vi "datataker.vi"() -> ()   [LabVIEW 2012]
doc: "This example demonstrates how to acquire a single buffer of voltage measurements using a DAQmx device.\n\nFor instructions on how to connect your signals to the DAQ device, refer to your device documentation."
uses:
  <vilib>/userdefined/High Color/nirio_resource_hc.ctl
  <vilib>/Utility/error.llb/DialogType.ctl
  <vilib>/FPGAPlugInAG/PCIe-7841R/niLvFpga_Open_PCIe-7841R.vi
  <vilib>/DAQmx/create/channels.llb/DAQmx Create Channel (AI-Voltage-Basic).vi
  <vilib>/DAQmx/configure/timing.llb/DAQmx Timing (Sample Clock).vi
  <vilib>/DAQmx/configure/trigger.llb/DAQmx Start Trigger (Digital Edge).vi
  <vilib>/rvi/interface/nirviOpenFPGA/nirviOpenFPGA.xnode
  fpga/MultiChannelFeed_FPGATarget2_feedbackcooling(_T5hmXv3JUos.lvbitx
  <resource>/objmgr/daqmx.rc
panel:
  in  "sweep time (S)":ext=10.0 format="%.2f"
  in  "sweep stop (Hz)":ext=200.0
  in  "sweep start (Hz)":ext=1.0
  in  "chirp?":bool
  in  "stop (F)":ext=200.0
  in  "start (F)":ext=10.0
  in  "Number of F Steps":i32=20
  in  "dc offset?":bool=TRUE
  in  "volt_div":dbl=200.0
  in  "Set synth?":bool=TRUE
  in  "stop (V)":ext=2.5
  in  "start (V)":ext=2.5
  in  "Number of V Steps":i32=1
  out "error out":errorcluster
  in  "Physical Channel (drive signals)":tag="Dev5/ai0"
  out "Curr threshold":dbl
  in  "Stop threshold":dbl=0.05
  in  "Stop flashing below thresh":bool
  out "Pirani pressure (mbar)":string="0000\r\n"
  out "CC read error":errorcluster={"status"=FALSE, "code"=1073676294, "source"="VISA Read in read_pressure(SubVI).vi->hdf5(SubVI).vi->datataker.vi"}
  out "CC pressure (mbar)":string="4."
  out "Pirani read error":errorcluster={"status"=FALSE, "code"=1073676294, "source"="VISA Read in read_pressure(SubVI).vi->hdf5(SubVI).vi->datataker.vi"}
  in  "# Pulses":i32=3
  in  "Output channel (for flashing)":tag="Dev4/ao0"
  in  "Number of cyles\nbetween flashes":i32=3
  in  "Flash lamp?":bool
  in  "File base name":string="5e-7mbar_xyzcool"
  in  "Delay time between files(s)":dbl caption="Delay Time (s)"
  in  "Num files":i32=100000
  out "Temps (C):":dbl[](array[numeric])=[24.1, 24.6]
  in  "VISA Refnum in":refnum<visa-resource-name>="GPIB0::19::INSTR"
  in  "RIO Device":T1="RIO0::INSTR"
  in  "Directory path":path=path "D:/Data/20140623/Bead1/freq_sweep_finer"
  out "Waveform Graph":dbl[][](graph)
  in  "Number of Samples":i32=500000
  in  "Sample Rate":dbl=5000.0
  in  "Sample Clock Source":tag="/Dev2/PXI_Clk10"
  in  "Terminal Configuration":i32(ring)=-1 items=["default"=-1, "RSE"=10083, "NRSE"=10078, "Differential"=10106, "Pseudodifferential"=12529]
  in  "Max Voltage":dbl=10.0
  in  "Physical Channels (Position signals)":tag="Dev2/ai0:7"
  out "Actual Sample Rate":dbl=5000.0 format="%0.2f"
  # "Channel Settings"
  # "Acquired Data"
  # "Timing Settings"
  # "Flash Lamp Settings"
  # "Pressures and Temperatures"
  # "Logging Settings"
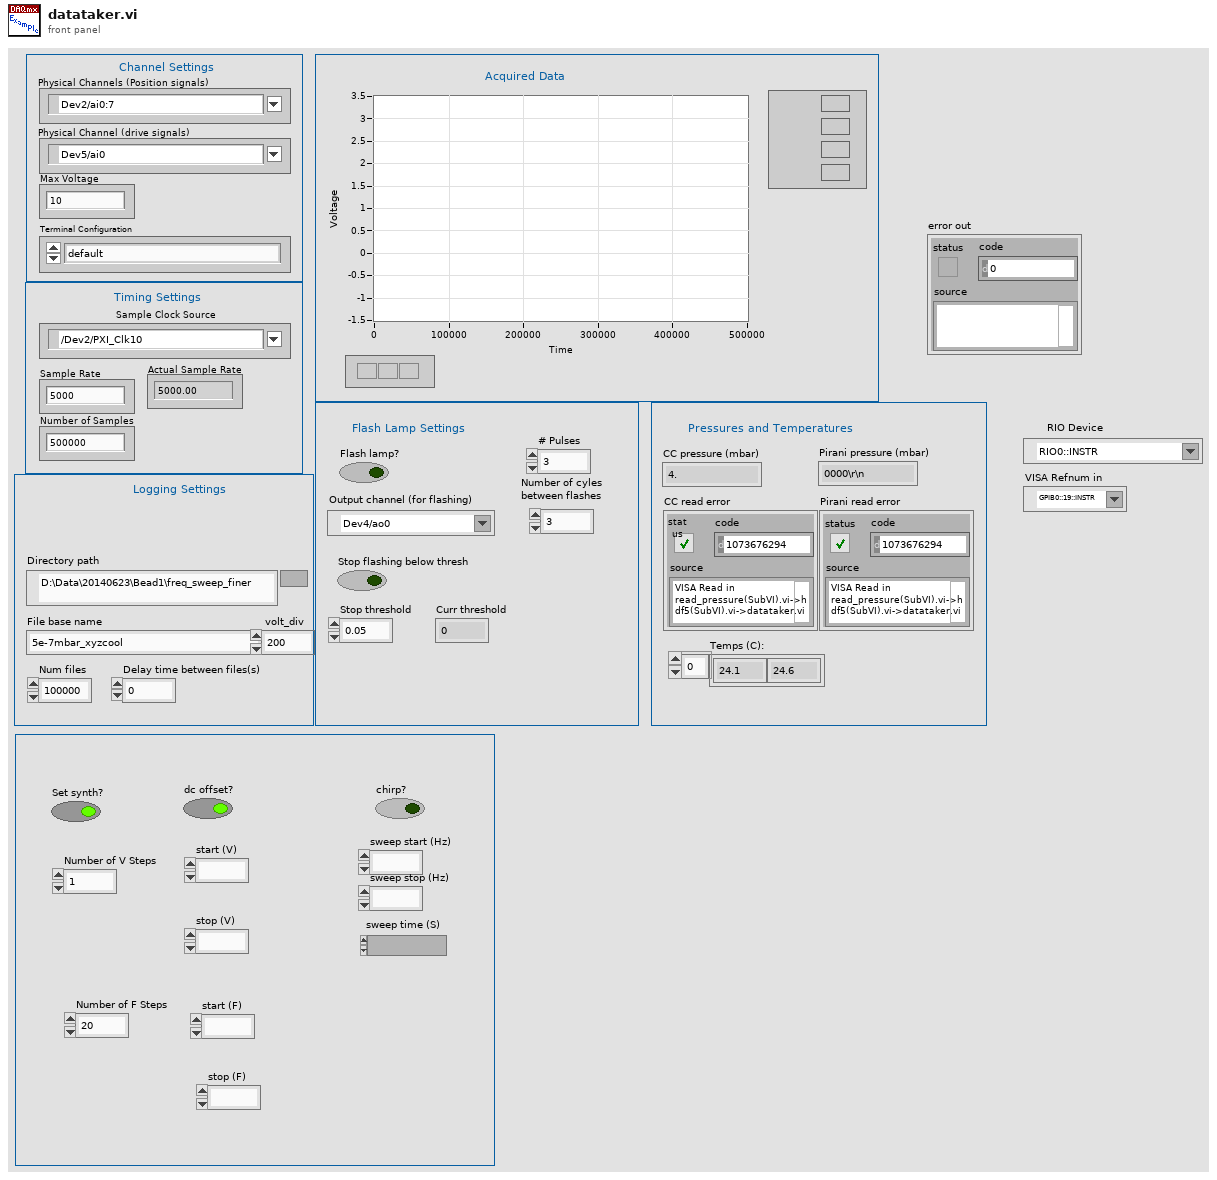
[diagram p1: front panel]
types:
  T1 = typedef "nirio_resource_hc.ctl" = tag
  T2 = typedef "DialogType.ctl" = u16
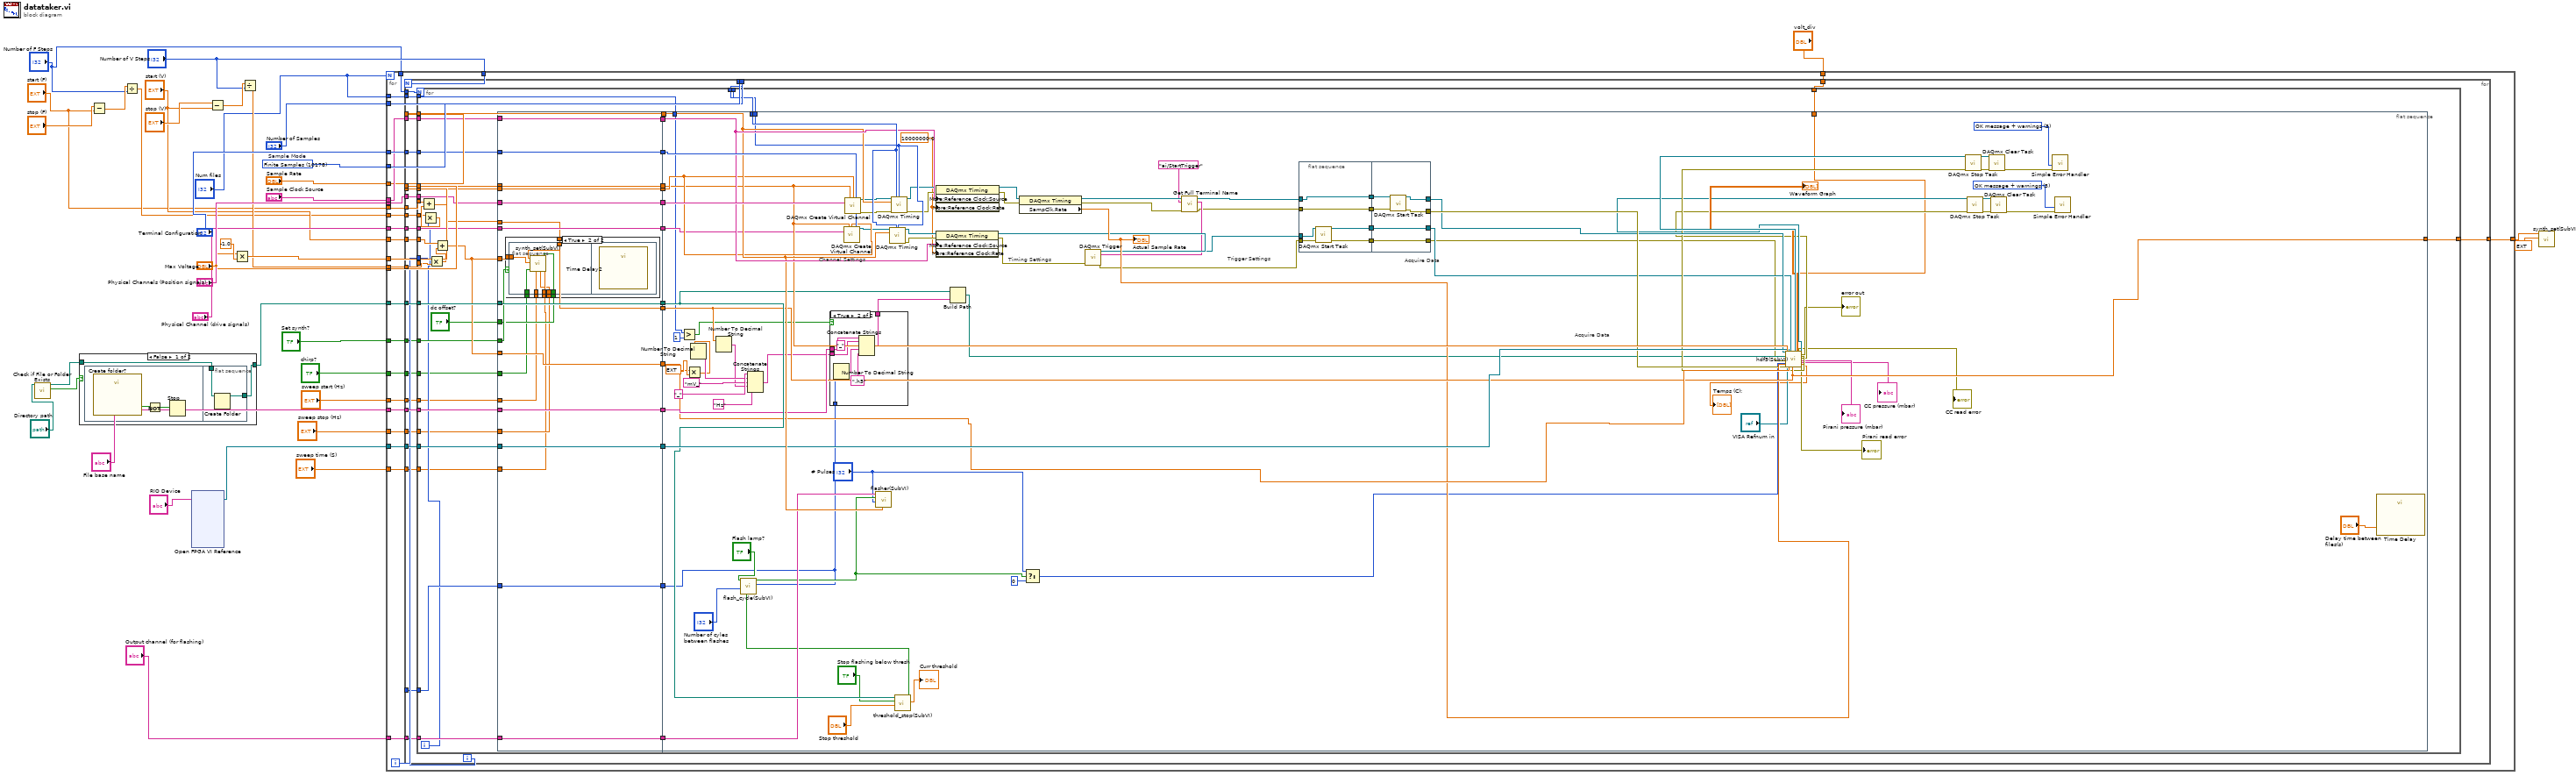
[diagram p0: block diagram]
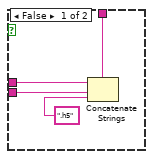
[diagram p3: hidden frame]
diagram:
  w37 = 10178 items=["Finite Samples"=10178, "Continuous Samples"=10123, "Hardware Timed Single Point"=12522]  # Sample Mode
  n1 = call <vilib>:"Check if File or Folder Exists.vi"("path"="Directory path") -> ("file or folder exists?"=w25:bool, "dup path"=w24:path)  [unwired: 8 in, 1 out]
  n2 = case shown="False" w25 {
    tunnel: w24 -> [w39 w44]
    tunnel: [w38 w44] -> w23
    frame False {
      n3 = flat-sequence {
        tunnel: w39 -> [w43]
        tunnel: [w42] -> w38
        frame #0 {
          n4 = call "Create folder?"() -> ("OK"=w41:bool)  [unwired: 18 in, 1 out]
          n5 = Not(x=w41) -> (.not. x?=w40:bool)
          n6 = Stop(stop? (T)=w40) -> ()
        }
        frame #1 {
          n7 = Create Folder(path (use dialog)=w43) -> (created path=w42:path)  [unwired: 2 in, 2 out]
        }
      }
    }
    frame True {
    }
  }
  n8 = Subtract(x="stop (F)", y="start (F)") -> (x-y=w9:ext)
  n9 = Divide(x=w9, y="Number of F Steps") -> (x/y=w8:ext)
  n10 = xnode "Open FPGA VI Reference"("resource name"="RIO Device") -> ("FPGA VI Reference Out"=w27:refnum<k20>)  [unwired: 1 in, 1 out]
  n11 = Subtract(x="stop (V)", y="start (V)") -> (x-y=w18:ext)
  n12 = Multiply(x="Max Voltage", y=-1.0) -> (x*y=w30:dbl)
  n13 = Divide(x=w18, y="Number of V Steps") -> (x/y=w16:ext)
  n14 = for {
    N: "Num files" -> [_]
    tunnel: w37 -> [w72]
    tunnel: "Physical Channels (Position signals)" -> [w71]
    tunnel: "Terminal Configuration" -> [w70]
    tunnel: "Sample Clock Source" -> [w69]
    tunnel: "Sample Rate" -> [w68]
    tunnel: "Number of Samples" -> [w67]
    tunnel: w30 -> [w66]
    tunnel: "Max Voltage" -> [w65]
    tunnel: w27 -> [w64]
    tunnel: w23 -> [w63]
    tunnel: "File base name" -> [w62]
    tunnel: "Output channel (for flashing)" -> [w61]
    tunnel: "Physical Channel (drive signals)" -> [w60]
    tunnel: "Number of V Steps" -> [w59]
    tunnel: w16 -> [w58]
    tunnel: "start (V)" -> [w57]
    tunnel: [w56] -> w6
    tunnel: "Num files" -> [w54]
    tunnel: "Set synth?" -> [w53]
    tunnel: "volt_div" -> [w52]
    tunnel: w8 -> [w51]
    tunnel: "start (F)" -> [w50]
    tunnel: "Number of F Steps" -> [w49]
    tunnel: "chirp?" -> [w48]
    tunnel: "sweep start (Hz)" -> [w47]
    tunnel: "sweep stop (Hz)" -> [w46]
    tunnel: "sweep time (S)" -> [w45]
    i -> [w55]
    n15 = for {
      N: w59 -> [_]
      tunnel: w72 -> [w100]
      tunnel: w71 -> [w99]
      tunnel: w70 -> [w98]
      tunnel: w69 -> [w97]
      tunnel: w68 -> [w96]
      tunnel: w67 -> [w95]
      tunnel: w66 -> [w94]
      tunnel: w65 -> [w93]
      tunnel: w64 -> [w92]
      tunnel: w63 -> [w91]
      tunnel: w62 -> [w90]
      tunnel: w61 -> [w89]
      tunnel: w60 -> [w88]
      tunnel: w58 -> [w87]
      tunnel: w57 -> [w86]
      tunnel: [w85] -> w56
      tunnel: w55 -> [w83]
      tunnel: w54 -> [w82]
      tunnel: w53 -> [w81]
      tunnel: w52 -> [w80]
      tunnel: w51 -> [w79]
      tunnel: w50 -> [w78]
      tunnel: w49 -> [w77]
      tunnel: w48 -> [w76]
      tunnel: w47 -> [w75]
      tunnel: w46 -> [w74]
      tunnel: w45 -> [w73]
      i -> [w84]
      n16 = for {
        N: w77 -> [_]
        tunnel: w100 -> [w133]
        tunnel: w99 -> [w132]
        tunnel: w98 -> [w131]
        tunnel: w97 -> [w130]
        tunnel: w96 -> [w129]
        tunnel: w95 -> [w128]
        tunnel: w94 -> [w127]
        tunnel: w93 -> [w126]
        tunnel: w92 -> [w125]
        tunnel: w91 -> [w124]
        tunnel: w90 -> [w123]
        tunnel: w89 -> [w122]
        tunnel: w88 -> [w121]
        tunnel: w87 -> [w120]
        tunnel: w86 -> [w118]
        tunnel: [w116] -> w85
        tunnel: w84 -> [w115]
        tunnel: w83 -> [w114]
        tunnel: w82 -> [w113]
        tunnel: w81 -> [w112]
        tunnel: w80 -> [w111]
        tunnel: w79 -> [w107]
        tunnel: w78 -> [w106]
        tunnel: w76 -> [w104]
        tunnel: w75 -> [w103]
        tunnel: w74 -> [w102]
        tunnel: w73 -> [w101]
        i -> [w105]
        n17 = Multiply(x=w107, y=w105) -> (x*y=w108:ext)
        n18 = Add(x=w106, y=w108) -> (x+y=w109:ext)
        n19 = Multiply(x=w115, y=w120) -> (x*y=w119:ext)
        n20 = Add(x=w118, y=w119) -> (x+y=w117:ext)
        n21 = flat-sequence {
          tunnel: w121 -> [w157]
          tunnel: w122 -> [w158]
          tunnel: w123 -> [w159]
          tunnel: w124 -> [w160]
          tunnel: w125 -> [w161]
          tunnel: w126 -> [w162]
          tunnel: w127 -> [w163]
          tunnel: w130 -> [w164]
          tunnel: w131 -> [w165]
          tunnel: w132 -> [w166]
          tunnel: [w166] -> w146
          tunnel: [w165] -> w145
          tunnel: [w164] -> w144
          tunnel: [w163] -> w143
          tunnel: [w162] -> w142
          tunnel: [w161] -> w141
          tunnel: [w160] -> w140
          tunnel: [w159] -> w139
          tunnel: [w158] -> w138
          tunnel: [w157] -> w137
          tunnel: w109 -> [w155]
          tunnel: w117 -> [w156]
          tunnel: [w155] -> w136
          tunnel: w117 -> [w154]
          tunnel: [w154] -> w135
          tunnel: w114 -> [w153]
          tunnel: [w153] -> w134
          tunnel: w112 -> [w152]
          tunnel: "dc offset?" -> [w151]
          tunnel: w104 -> [w150]
          tunnel: w103 -> [w149]
          tunnel: w102 -> [w148]
          tunnel: w101 -> [w147]
          tunnel: w133 -> [w270]
          tunnel: w129 -> [w266]
          tunnel: w128 -> [w265]
          tunnel: w146 -> [w269]
          tunnel: w145 -> [w268]
          tunnel: w144 -> [w267]
          tunnel: w143 -> [w264]
          tunnel: w142 -> [w263]
          tunnel: w141 -> [w262]
          tunnel: w140 -> [w261]
          tunnel: w139 -> [w260]
          tunnel: w138 -> [w259]
          tunnel: w137 -> [w258]
          tunnel: w136 -> [w256]
          tunnel: w135 -> [w257]
          tunnel: [w256] -> w116
          tunnel: w134 -> [w183]
          tunnel: w113 -> [w182]
          tunnel: w111 -> [w181]
          frame #0 {
            n22 = case shown="True" w152 {
              tunnel: w156 -> [_ w173]
              tunnel: w155 -> [_ w172]
              tunnel: w151 -> [_ w171]
              tunnel: w150 -> [_ w170]
              tunnel: w149 -> [_ w169]
              tunnel: w148 -> [_ w168]
              tunnel: w147 -> [_ w167]
              frame False {
              }
              frame True {
                n23 = flat-sequence {
                  tunnel: w173 -> [w180]
                  tunnel: w172 -> [w179]
                  tunnel: w171 -> [w178]
                  tunnel: w170 -> [w177]
                  tunnel: w169 -> [w176]
                  tunnel: w168 -> [w174]
                  tunnel: w167 -> [w175]
                  frame #0 {
                    n24 = call "synth_set(SubVI).vi"("sweep time (S)"=w175, "dc offset?"=w178, "sweep stop (Hz)"=w174, "sweep start (Hz)"=w176, "chirp?"=w177, "amplitude (V)"=w180, "frequency (Hz)"=w179) -> ()  [unwired: 5 in]
                  }
                  frame #1 {
                    n25 = call "Time Delay2"() -> ()  [unwired: 11 in, 1 out]
                  }
                }
              }
            }
          }
          frame #1 {
            w201 = 10000000.0 ("RefClk.Rate")
            w204 = T2 3 items=["no dialog", "OK message", "continue or stop message", "OK message + warnings", "continue/stop + warnings"] ("type of dialog (OK msg:1)")
            w248 = T2 3 items=["no dialog", "OK message", "continue or stop message", "OK message + warnings", "continue/stop + warnings"] ("type of dialog (OK msg:1)")
            # "Acquire Data"
            # "Acquire Data"
            # "Trigger Settings"
            # "Timing Settings"
            # "Channel Settings"
            n26 = Greater?(x=w182, y=1) -> (0:w240:bool)
            n27 = Multiply(x=ext 1000.0, y=w257) -> (x*y=w184:ext)
            n28 = Number To Decimal String(number=w184) -> (decimal integer string=w190:string)  [unwired: 1 in]
            n29 = Number To Decimal String(number=w256) -> (decimal integer string=w188:string)  [unwired: 1 in]
            n30 = Concatenate Strings("_" ("string"), w190, "mV_" ("string"), w188, "Hz" ("string")) -> (w186:string)
            n31 = case shown="True" w240 {
              tunnel: w183 -> [_ w291]
              tunnel: [w285 w289] -> w238
              tunnel: w186 -> [w284 w287]
              tunnel: w260 -> [w283 w288]
              frame False {
                n32 = Concatenate Strings(w283, w284, ".h5" ("string")) -> (w285:string)
              }
              frame True {
                n33 = Number To Decimal String(number=w291) -> (decimal integer string=w292:string)  [unwired: 1 in]
                n34 = Concatenate Strings(w288, w287, "_" ("string"), w292, ".h5" ("string")) -> (w289:string)
              }
            }
            n35 = call-poly <vilib>:"DAQmx Create Virtual Channel.vi"("maximum value"=w263, "minimum value"=w264, "input terminal configuration"=w268, "physical channels"=w258) -> ("task out"=w227:refnum<k21>)  [unwired: 10 in, 1 out]
            n36 = call-poly <vilib>:"DAQmx Create Virtual Channel.vi"("maximum value"=w263, "minimum value"=w264, "input terminal configuration"=w268, "physical channels"=w269) -> ("task out"=w229:refnum<k21>, "error out"=w228:errorcluster)  [unwired: 10 in]
            n37 = call-poly <vilib>:"DAQmx Timing.vi"("task/channels in"=w227, "sample mode"=w270, "samples per channel"=w265, "rate"=w266) -> ("task out"=w224:refnum<k21>, "error out"=w223:errorcluster)  [unwired: 10 in]
            n38 = call-poly <vilib>:"DAQmx Timing.vi"("task/channels in"=w229, "sample mode"=w270, "samples per channel"=w265, "rate"=w266, "error in"=w228) -> ("task out"=w226:refnum<k21>, "error out"=w225:errorcluster)  [unwired: 9 in]
            n39 = call "threshold_stop(SubVI).vi"("Stop threshold"="Stop threshold", "Stop flashing below thresh"="Stop flashing below thresh", "dup path"=w261) -> ("Curr threshold"=→"Curr threshold":dbl, "Boolean"=w234:bool)  [unwired: 7 in]
            n40 = call "flash_cycle(SubVI).vi"("Boolean in"=w234, "Number of cyles\nbetween flashes"="Number of cyles\nbetween flashes", "Numeric"=w183, "Flash lamp?"="Flash lamp?") -> ("Boolean out"=w233:bool)  [unwired: 7 in]
            n41 = call "flasher(SubVI).vi"("Sample Rate"=w266, "# Pulses"="# Pulses", "Boolean"=w233, "Output channel (for flashing)"=w259) -> ()  [unwired: 8 in]
            n42 = property class="DAQmx Timing"(reference=w224, error in=w223, "More:Reference Clock:Source"=w267, "More:Reference Clock:Rate"=w201) -> (reference out=w217:refnum<k21>, error out=w216:errorcluster)
            n43 = property class="DAQmx Timing"(reference=w226, error in=w225, "More:Reference Clock:Source"=w267, "More:Reference Clock:Rate"=w201) -> (reference out=w222:refnum<k21>, error out=w221:errorcluster)
            n44 = Build Path(base path=w261, name or relative path=w238) -> (appended path=w239:path)
            n45 = property class="DAQmx Timing"(reference=w222, error in=w221) -> (reference out=w220:refnum<k21>, error out=w218:errorcluster, "SampClk.Rate"=w247:dbl)
            "Actual Sample Rate" <- w247
            n46 = Select(t="# Pulses", s=w233, f=0) -> (s? t:f=w230:i32)
            n47 = call "Get Full Terminal Name.vi"("error in"=w218, "Local Terminal Name"="ai/StartTrigger", "task/channels in"=w220) -> ("error out"=w213:errorcluster, "Terminal Name with Device Prefix"=w215:tag, "task out"=w214:refnum<k21>)  [unwired: 6 in]
            n48 = call-poly <vilib>:"DAQmx Trigger.vi"("task/channels in"=w217, "source"=w215, "error in"=w216) -> ("task out"=w212:refnum<k21>, "error out"=w211:errorcluster)  [unwired: 11 in]
            n49 = flat-sequence {
              tunnel: w214 -> [w274]
              tunnel: w213 -> [w273]
              tunnel: w212 -> [w276]
              tunnel: w211 -> [w275]
              tunnel: [w274] -> w255
              tunnel: [w273] -> w254
              tunnel: [w272] -> w253
              tunnel: [w271] -> w252
              tunnel: [w281] -> w245
              tunnel: [w279] -> w246
              tunnel: w255 -> [w282]
              tunnel: w254 -> [w280]
              tunnel: [w278] -> w210
              tunnel: w253 -> [w278]
              tunnel: [w277] -> w209
              tunnel: w252 -> [w277]
              frame #0 {
                n50 = call <vilib>:"DAQmx Start Task.vi"("task/channels in"=w276, "error in"=w275) -> ("task out"=w272:refnum<k21>, "error out"=w271:errorcluster)  [unwired: 12 in]
              }
              frame #1 {
                n51 = call <vilib>:"DAQmx Start Task.vi"("task/channels in"=w282, "error in"=w280) -> ("task out"=w281:refnum<k21>, "error out"=w279:errorcluster)  [unwired: 12 in]
              }
            }
            n52 = call "hdf5(SubVI).vi"("Refnum in"=w245, "VISA Refnum in"="VISA Refnum in", "appended path"=w239, "Max Voltage"=w263, "error out 3"=w209, "f"=w230, "SampClk.Rate"=w247, "error in (no error)"=w246, "FPGA VI Reference Out"=w262, "drive_amplitude"=w257, "task in"=w210, "drive_freq"=w256, "volt_div"=w181) -> ("task out 4"=w244:refnum<k21>, "Array"=→"Waveform Graph":dbl[][], "CC read error"=→"CC read error":errorcluster, "Refnum out"=w203:refnum<k21>, 21:"error out"=→"error out":errorcluster, "error out 4"=w243:errorcluster, "error out 2"=w202:errorcluster, "Pirani pressure (mbar)"=→"Pirani pressure (mbar)":string, "CC pressure (mbar)"=→"CC pressure (mbar)":string, "Temps (C):"=→"Temps (C):":dbl[], 27:"error out"=→"Pirani read error":errorcluster)  [unwired: 4 in]
            n53 = call <vilib>:"DAQmx Stop Task.vi"("task/channels in"=w244, "error in"=w243) -> ("task out"=w250:refnum<k21>, "error out"=w249:errorcluster)  [unwired: 12 in]
            n54 = call <vilib>:"DAQmx Stop Task.vi"("task/channels in"=w203, "error in"=w202) -> ("task out"=w206:refnum<k21>, "error out"=w205:errorcluster)  [unwired: 12 in]
            n55 = call <vilib>:"DAQmx Clear Task.vi"("task in"=w250, "error in"=w249) -> ("error out"=w251:errorcluster)  [unwired: 13 in]
            n56 = call <vilib>:"DAQmx Clear Task.vi"("task in"=w206, "error in"=w205) -> ("error out"=w207:errorcluster)  [unwired: 13 in]
            n57 = call <vilib>:"Simple Error Handler.vi"("type of dialog (OK msg:1)"=w248, "error in (no error)"=w251) -> ()  [unwired: 3 in, 5 out]
            n58 = call <vilib>:"Simple Error Handler.vi"("type of dialog (OK msg:1)"=w204, "error in (no error)"=w207) -> ()  [unwired: 3 in, 5 out]
            n59 = call "Time Delay"("Delay Time (s)"="Delay time between files(s)") -> ()  [unwired: 10 in, 1 out]
          }
        }
      }
    }
  }
  n60 = call "synth_set(SubVI).vi"("amplitude (V)"=ext 0.00099999999999999999996, "frequency (Hz)"=w6) -> ()  [unwired: 10 in]
